vi "A170316-11-Main-large.vi"() -> ()   [LabVIEW 2020]
uses:
  System.Windows.Forms
  Database/Global1.vi
  Global_Variable/Global.vi
  <userlib>/_MGI/Menu Building/MenuItemStatusChange/MGI_MenuItemStatusChange.lvclass
panel:
  out "前序状态字":string
  out "前序状态":bool
  out "ECU自动":bool
  out "电机结果显示":string
  in  "质量报警":bool caption="布尔"
  in  "设备缺料":bool caption="布尔"
  in  "设备故障":bool caption="布尔"
  in  "设备离线":bool caption="布尔"
  in  "设备正常":bool caption="布尔"
  in  "菜单":refnum<k24>(container)
  out "检测结果":bool
  in  "批次信息":string[][](table)
  out "提示信息":string
  out "错误":bool
  out "时间字符串":string
  out "日期字符串":string
  out "电机自动":bool
  out "userStatus":string caption="用户状态"
  out "userName":string caption="用户名"
  out "生产数量":u32
  out "追溯码":string
  out "connectionMode":string caption="联机类型"
  out "产品型号":string
  in  "更换产品":refnum<vi>
  # "激光打标机"
  # "打标结果"
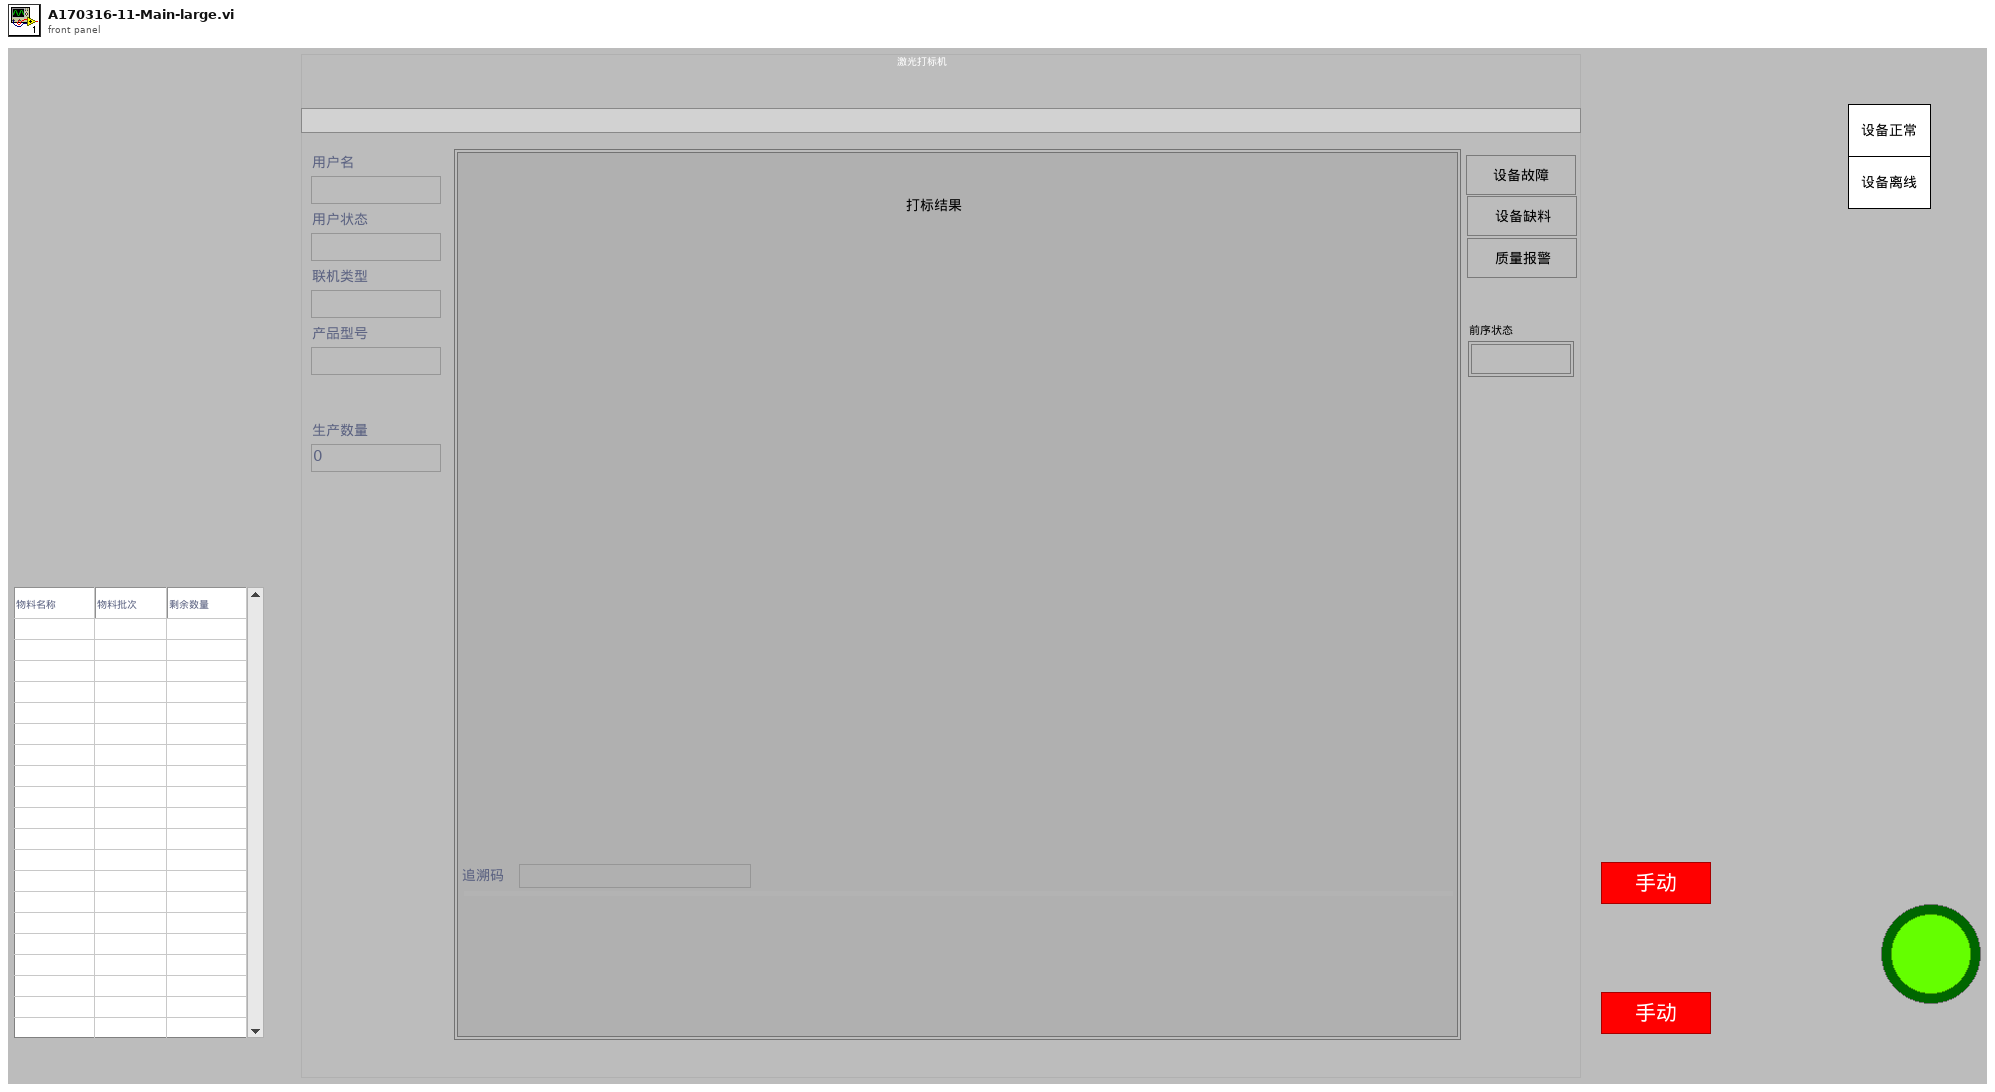
[diagram p1: front panel]
types:
  T1 = enum32{"Invalid", "Standard", "Closed", "Hidden", "Minimized", "Maximized"}
  T2 = enum32{"invalid app kind", "Development System", "Run Time System", "Student Edition", "Embedded LabVIEW", "Evaluation", "Custom"}
  T3 = cluster{"Core":cluster{"Current VI Reference":refnum<vi>, "Close Panel on Exit?":bool}, "Your Boolean data":bool, "Your string data":string}
  T4 = cluster{"Current VI Reference":refnum<vi>, "Close Panel on Exit?":bool}
  T5 = cluster{"用户编号":string, "用户名":string, "用户密码(密文)":string, "用户权限":string}
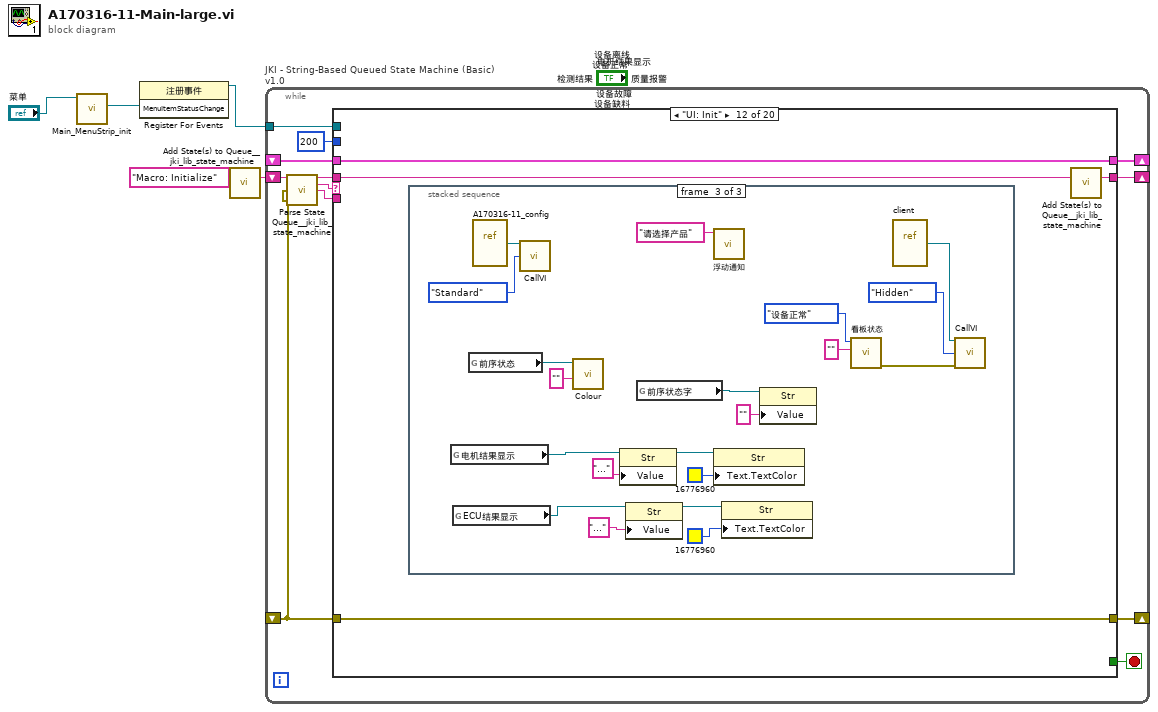
[diagram p0: block diagram]
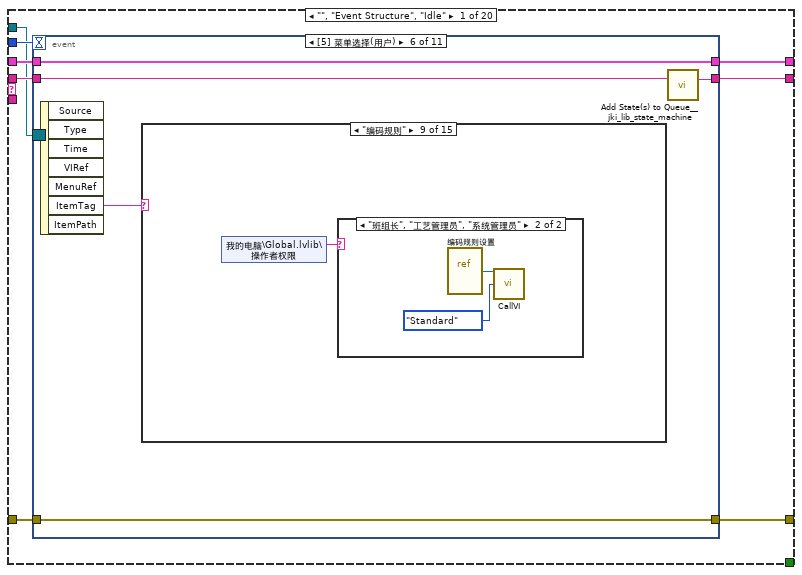
[diagram p2: hidden frame]
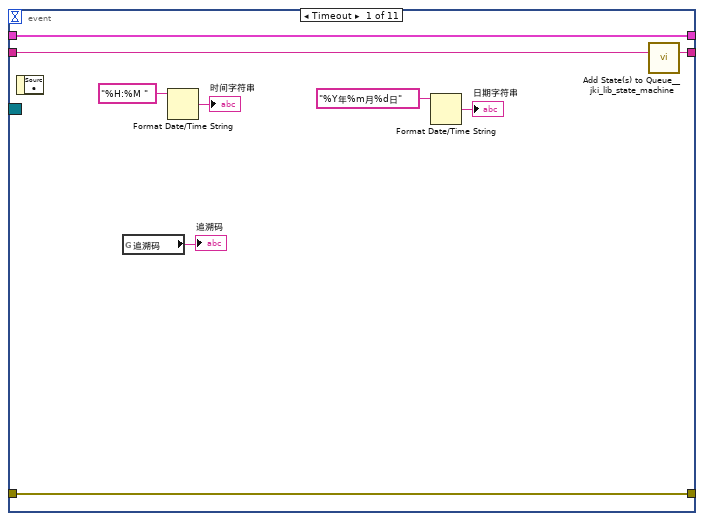
[diagram p3: hidden frame]
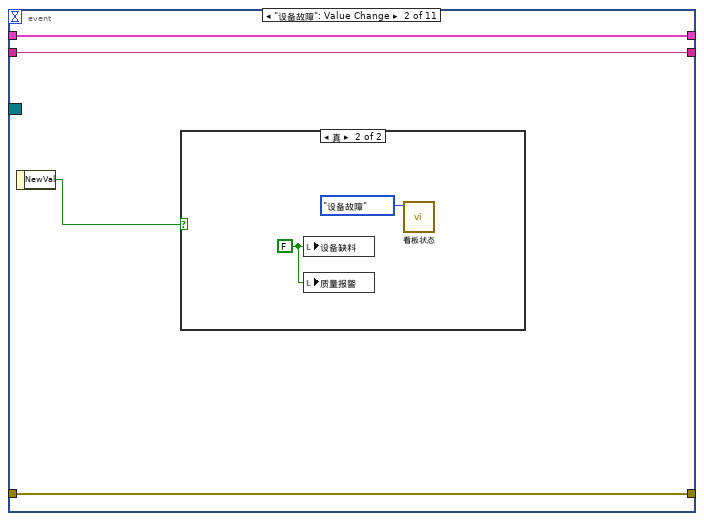
[diagram p4: hidden frame]
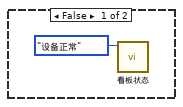
[diagram p5: hidden frame]
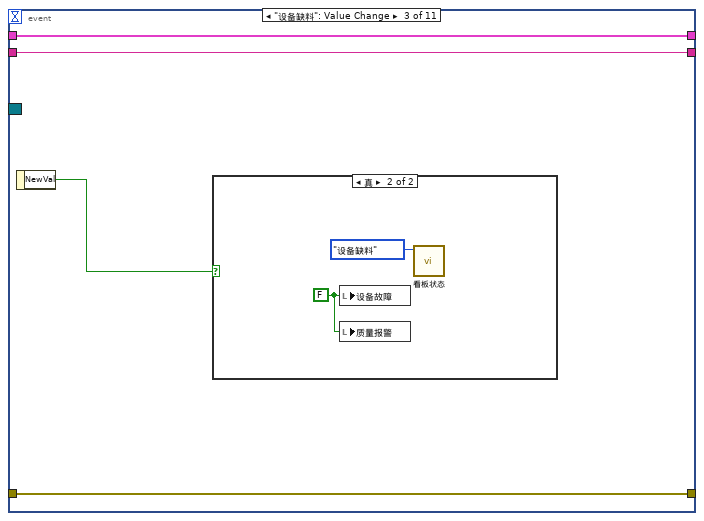
[diagram p6: hidden frame]
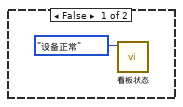
[diagram p7: hidden frame]
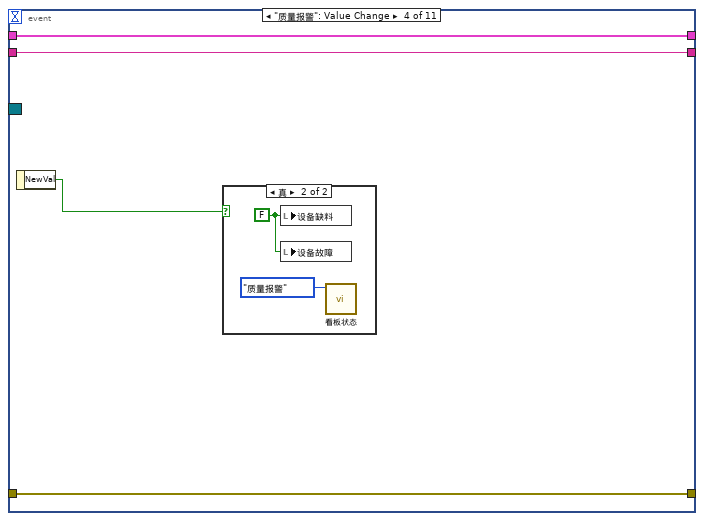
[diagram p8: hidden frame]
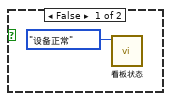
[diagram p9: hidden frame]
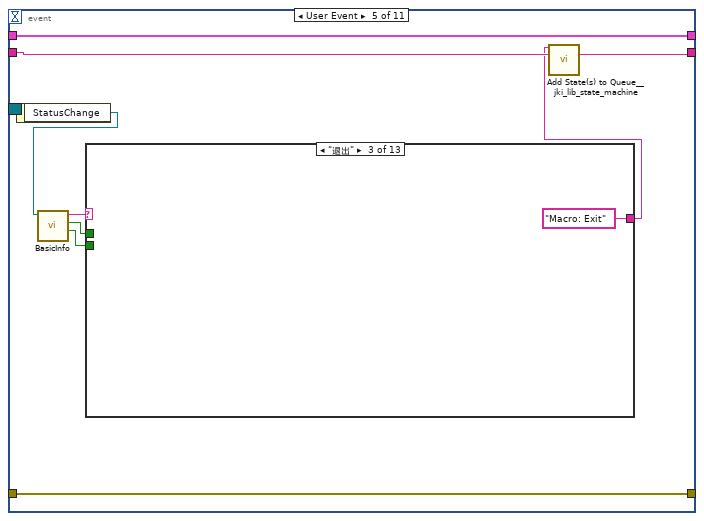
[diagram p10: hidden frame]
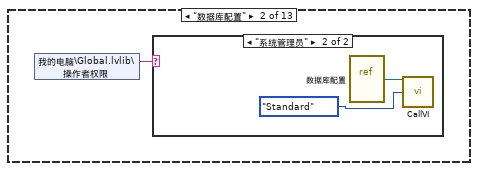
[diagram p12: hidden frame]
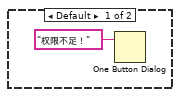
[diagram p13: hidden frame]
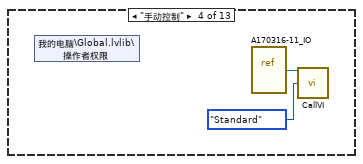
[diagram p14: hidden frame]
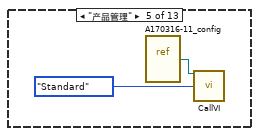
[diagram p15: hidden frame]
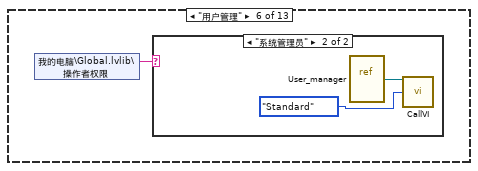
[diagram p16: hidden frame]
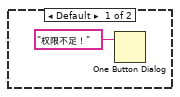
[diagram p17: hidden frame]
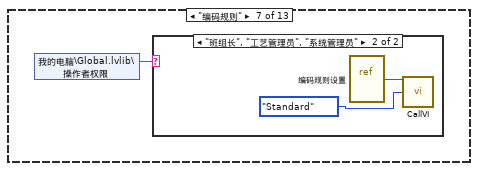
[diagram p18: hidden frame]
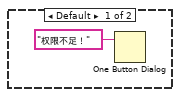
[diagram p19: hidden frame]
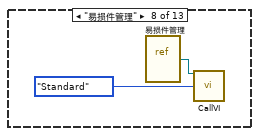
[diagram p20: hidden frame]
diagram:
  n1 = call "Main_MenuStrip_init.vi"("MenuStrip"="菜单") -> ("MenuItemStatusChange"=w2:refnum<user-event>)  [unwired: 9 in, 1 out]
  n2 = register-events(w2) -> (reference out=w1:refnum<event-registration>)  [unwired: 2 in, 1 out]
  n3 = call <vilib>:"Add State(s) to Queue__jki_lib_state_machine.vi"("State(s) in (\"\")"="Macro: Initialize") -> ("States Out"=w5:string)  [unwired: 14 in]
  n4 = while "JKI - String-Based Queued State Machine (Basic) v1.0" {
    shift-right: [w10] -> _
    shift-left: _ -> [w9]
    shift-right: [w13] -> _
    shift-left: _ -> [w7]
    shift-right: [w12] -> _
    shift-left: w5 -> [w14]
    tunnel: w1 -> [w6]
    stop <- w11 stop-if-true
    n5 = call <vilib>:"Parse State Queue__jki_lib_state_machine.vi"("State Queue"=w14, "Error In (no error)"=w7) -> ("Remaining States"=w16:string, "Current State"=w17:string, "Arguments"=w15:string)  [unwired: 11 in]
    n6 = case shown="\"UI: Init\"" w17 {
      selector: w17 -> [_ _ w202 _ _ _ _ _ _ _ _ _ _ _ _ _ _ _ _ _]
      tunnel: w16 -> [w25 w201 w206 w224 w230 w235 w239 w246 w252 w256 w268 w272 w319 w330 w356 w361 w374 w378 w382 w386]
      tunnel: w15 -> [_ _ _ _ _ _ _ _ _ _ _ _ w314 w324 _ _ _ _ _ _]
      tunnel: w9 -> [w23 w198 w204 w215 w227 w233 w236 _ w247 w253 w266 w270 w317 w326 w353 w358 w371 w375 w379 w383]
      tunnel: [w22 w199 w208 w221 errorcluster {"status"=FALSE, "code"=0, "source"=""} ("error out") w232 w237 w243 w248 w254 w263 w269 w315 w327 w354 w359 w372 w376 w380 w384] -> w13
      tunnel: w7 -> [w21 w199 w207 w221 w226 w232 w237 w243 w249 w254 w258 w269 w316 w328 w354 w359 w372 w376 w380 w384]
      tunnel: [w24 w200 w205 w223 w229 w234 w238 w245 w251 w255 w267 w271 w318 w329 w355 w360 w373 w377 w381 w385] -> w12
      tunnel: [_ _ _ _ _ TRUE _ _ _ _ _ _ _ _ _ _ _ _ _ _] -> w11
      tunnel: [w20 w198 w204 w222 w227 w233 w236 w244 w247 w253 w266 w270 w317 w326 w353 w358 w371 w375 w379 w383] -> w10
      tunnel: 200 ("Timeout") -> [w19 _ _ _ _ _ _ _ _ _ _ _ _ _ _ _ _ _ _ _]
      tunnel: w6 -> [w18 _ _ _ _ _ _ _ _ _ _ _ _ _ _ _ _ _ _ _]
      frame "", "Event Structure", "Idle" {
        n7 = event shown="[5] 菜单选择(用户)" {
          selector: w18 -> [_ _ _ _ _ _ _ _ _ _ _]
          dyn-events: _ -> [_ _ _ _ _ _ _ _ _ _ _]
          timeout: w19 -> [_ _ _ _ _ _ _ _ _ _ _]
          tunnel: w25 -> [w34 w37 w44 w51 w59 w105 w155 w161 w182 w191 w194]
          tunnel: [w33 w37 w44 w51 w58 w103 w156 w161 w182 w190 w195] -> w24
          tunnel: w23 -> [w31 w38 w45 w52 w60 w104 w157 w162 w183 w188 w197]
          tunnel: [w32 w36 w43 w50 w56 w106 w154 w160 w181 w189 w196] -> w22
          tunnel: w21 -> [w32 w36 w43 w50 w56 w106 w154 w160 w181 w189 w196]
          tunnel: [w31 w38 w45 w52 w60 w104 w157 w162 w183 w188 w197] -> w20
          event Timeout {
            n8 = event-data() -> ()  [unwired: 1 in, 1 out]
            n9 = global read "Global1.vi" "追溯码"() -> (→"追溯码":string)
            n10 = Format Date/Time String(time format string (%c)="%H:%M ") -> (date/time string=→"时间字符串":string)  [unwired: 2 in]
            n11 = Format Date/Time String(time format string (%c)="%Y年%m月%d日") -> (date/time string=→"日期字符串":string)  [unwired: 2 in]
            n12 = call <vilib>:"Add State(s) to Queue__jki_lib_state_machine.vi"("State(s) in (\"\")"=w34) -> ("States Out"=w33:string)  [unwired: 14 in]
          }
          event "设备故障": Value Change {
            n13 = event-data() -> ("NewVal"=w35:bool)  [unwired: 1 in]
            n14 = case shown="真" w35 {
              frame False {
                n15 = call "看板状态.vi"("设备状态"=enum16{"设备离线", "设备正常", "设备缺料", "设备故障", "质量报警"}."设备正常") -> ()  [unwired: 10 in, 1 out]
              }
              frame True {
                w40 = FALSE ("质量报警")
                n16 = local write "设备缺料"(w40) -> ()
                n17 = local write "质量报警"(w40) -> ()
                n18 = call "看板状态.vi"("设备状态"=enum16{"设备离线", "设备正常", "设备缺料", "设备故障", "质量报警"}."设备故障") -> ()  [unwired: 10 in, 1 out]
              }
            }
          }
          event "设备缺料": Value Change {
            n19 = event-data() -> ("NewVal"=w42:bool)  [unwired: 1 in]
            n20 = case shown="真" w42 {
              frame False {
                n21 = call "看板状态.vi"("设备状态"=enum16{"设备离线", "设备正常", "设备缺料", "设备故障", "质量报警"}."设备正常") -> ()  [unwired: 10 in, 1 out]
              }
              frame True {
                w47 = FALSE ("质量报警")
                n22 = local write "设备故障"(w47) -> ()
                n23 = local write "质量报警"(w47) -> ()
                n24 = call "看板状态.vi"("设备状态"=enum16{"设备离线", "设备正常", "设备缺料", "设备故障", "质量报警"}."设备缺料") -> ()  [unwired: 10 in, 1 out]
              }
            }
          }
          event "质量报警": Value Change {
            n25 = event-data() -> ("NewVal"=w49:bool)  [unwired: 1 in]
            n26 = case shown="真" w49 {
              frame False {
                n27 = call "看板状态.vi"("设备状态"=enum16{"设备离线", "设备正常", "设备缺料", "设备故障", "质量报警"}."设备正常") -> ()  [unwired: 10 in, 1 out]
              }
              frame True {
                w54 = FALSE ("质量报警")
                n28 = local write "设备缺料"(w54) -> ()
                n29 = local write "设备故障"(w54) -> ()
                n30 = call "看板状态.vi"("设备状态"=enum16{"设备离线", "设备正常", "设备缺料", "设备故障", "质量报警"}."质量报警") -> ()  [unwired: 10 in, 1 out]
              }
            }
          }
          event User Event {
            n31 = event-data() -> ("StatusChange"=w61:refnum<class "MGI_MenuItemStatusChange.lvclass">)  [unwired: 1 in]
            n32 = call <userlib>:"BasicInfo.vi"("MGI_MenuItemStatusChange in"=w61) -> ("Enabled?"=w64:bool, "Checked?"=w63:bool, "Tag"=w62:string)  [unwired: 7 in, 1 out]
            n33 = case shown="\"退出\"" w62 {
              tunnel: w63 -> [_ _ _ _ _ _ _ _ _ _ _ _ _]
              tunnel: w64 -> [_ _ _ _ _ _ _ _ _ _ _ _ _]
              tunnel: [_ _ "Macro: Exit" _ _ _ _ _ _ _ _ _ _] -> w57
              frame Default {
              }
              frame "数据库配置" {
                n34 = shared-variable "我的电脑\\Global.lvlib\\操作者权限"() -> (w65:string)  [unwired: 1 in, 1 out]
                n35 = case shown="\"系统管理员\"" w65 {
                  frame Default {
                    n36 = One Button Dialog(message="权限不足！" ("消息")) -> ()  [unwired: 1 in, 1 out]
                  }
                  frame "系统管理员" {
                    n37 = vi-ref "数据库配置.vi"() -> (w68:refnum<vi>)
                    n38 = call "CallVI.vi"("VI引用"=w68, "状态"=T1."Standard") -> ()  [unwired: 11 in, 3 out]
                  }
                }
              }
              frame "退出" {
              }
              frame "手动控制" {
                n39 = shared-variable "我的电脑\\Global.lvlib\\操作者权限"() -> ()  [unwired: 1 in, 2 out]
                n40 = vi-ref "A170316-11_IO.vi"() -> (w71:refnum<vi>)
                n41 = call "CallVI.vi"("VI引用"=w71, "状态"=T1."Standard") -> ()  [unwired: 11 in, 3 out]
              }
              frame "产品管理" {
                n42 = vi-ref "A170316-11_config.vi"() -> (w73:refnum<vi>)
                n43 = call "CallVI.vi"("VI引用"=w73, "状态"=T1."Standard") -> ()  [unwired: 11 in, 3 out]
              }
              frame "用户管理" {
                n44 = shared-variable "我的电脑\\Global.lvlib\\操作者权限"() -> (w74:string)  [unwired: 1 in, 1 out]
                n45 = case shown="\"系统管理员\"" w74 {
                  frame Default {
                    n46 = One Button Dialog(message="权限不足！" ("消息")) -> ()  [unwired: 1 in, 1 out]
                  }
                  frame "系统管理员" {
                    n47 = vi-ref "User_manager.vi"() -> (w77:refnum<vi>)
                    n48 = call "CallVI.vi"("VI引用"=w77, "状态"=T1."Standard") -> ()  [unwired: 11 in, 3 out]
                  }
                }
              }
              frame "编码规则" {
                n49 = shared-variable "我的电脑\\Global.lvlib\\操作者权限"() -> (w78:string)  [unwired: 1 in, 1 out]
                n50 = case shown="\"班组长\", \"工艺管理员\", \"系统管理员\"" w78 {
                  frame Default {
                    n51 = One Button Dialog(message="权限不足！" ("消息")) -> ()  [unwired: 1 in, 1 out]
                  }
                  frame "班组长", "工艺管理员", "系统管理员" {
                    n52 = vi-ref "编码规则设置.vi"() -> (w81:refnum<vi>)
                    n53 = call "CallVI.vi"("VI引用"=w81, "状态"=T1."Standard") -> ()  [unwired: 11 in, 3 out]
                  }
                }
              }
              frame "易损件管理" {
                n54 = vi-ref "易损件管理.vi"() -> (w83:refnum<vi>)
                n55 = call "CallVI.vi"("VI引用"=w83, "状态"=T1."Standard") -> ()  [unwired: 11 in, 3 out]
              }
              frame "物料批次管理" {
                n56 = vi-ref "批次管理.vi"() -> (w85:refnum<vi>)
                n57 = call "CallVI.vi"("VI引用"=w85, "状态"=T1."Standard") -> ()  [unwired: 11 in, 3 out]
              }
              frame "报表" {
                n58 = call "文件对话框2"("start path"=path "D:/report", "prompt"="打开报表", "pattern (all files)"="*.doc;*.docx", "pattern label"="Word 文档") -> ("selected path"=w86:path, "error out"=w87:errorcluster)  [unwired: 8 in, 2 out]
                n59 = case shown="无错误" w87 {
                  selector: w87 -> [w93 w95]
                  tunnel: w86 -> [w94 _]
                  frame No Error {
                    w92 = 1 items=["Normal", "Maximize", "Minimize"] ("cpubbs_WindowState")
                    n60 = call "Open_Word.vi"("File Path"=w94, "cpubbs_WindowState"=w92, "错误输入（无错误）"=w93) -> ()  [unwired: 12 in, 1 out]
                  }
                  frame Error {
                    n61 = call <vilib>:"Clear Errors.vi"("error in (no error)"=w95) -> ()  [unwired: 5 in, 2 out]
                  }
                }
              }
              frame "报警信息" {
                n62 = vi-ref "报警信息.vi"() -> (w97:refnum<vi>)
                n63 = call "CallVI.vi"("VI引用"=w97, "状态"=T1."Standard") -> ()  [unwired: 11 in, 3 out]
              }
              frame "关于" {
                n64 = vi-ref "About.vi"() -> (w99:refnum<vi>)
                n65 = call "CallVI.vi"("VI引用"=w99, "状态"=T1."Standard") -> ()  [unwired: 11 in, 3 out]
              }
              frame "操作演示" {
                n66 = call <vilib>:"Application Directory.vi"() -> ("Application Directory"=w102:path)
                n67 = Build Path(base path=w102, name or relative path="操作演示" ("名称或相对路径")) -> (appended path=w101:path)
                n68 = call "自动播放ppt.vi"("路径"=w101) -> ()  [unwired: 10 in, 1 out]
              }
            }
            n69 = call <vilib>:"Add State(s) to Queue__jki_lib_state_machine.vi"("State(s) in Front (\"\")"=w57, "State(s) in (\"\")"=w59) -> ("States Out"=w58:string)  [unwired: 13 in]
          }
          event Menu Selection (User) {
            n70 = event-data() -> ("ItemTag"=w107:string)  [unwired: 1 in, 6 out]
            n71 = case shown="\"编码规则\"" w107 {
              frame "假", Default {
              }
              frame "数据库配置" {
                n72 = shared-variable "我的电脑\\Global.lvlib\\操作者权限"() -> (w108:string)  [unwired: 1 in, 1 out]
                n73 = case shown="\"系统管理员\"" w108 {
                  frame Default {
                    n74 = One Button Dialog(message="权限不足！" ("消息")) -> ()  [unwired: 1 in, 1 out]
                  }
                  frame "系统管理员" {
                    n75 = vi-ref "数据库配置.vi"() -> (w111:refnum<vi>)
                    n76 = call "CallVI.vi"("VI引用"=w111, "状态"=T1."Standard") -> ()  [unwired: 11 in, 3 out]
                  }
                }
              }
              frame "退出" {
                n77 = Quit LabVIEW() -> ()  [unwired: 1 in]
              }
              frame "手动控制" {
                n78 = shared-variable "我的电脑\\Global.lvlib\\操作者权限"() -> (w112:string)  [unwired: 1 in, 1 out]
                n79 = case shown="\"班组长\", \"系统管理员\"" w112 {
                  frame Default {
                    n80 = One Button Dialog(message="权限不足！" ("消息")) -> ()  [unwired: 1 in, 1 out]
                  }
                  frame "班组长", "系统管理员" {
                    n81 = vi-ref "A170316-11_IO.vi"() -> (w115:refnum<vi>)
                    n82 = call "CallVI.vi"("VI引用"=w115, "状态"=T1."Standard") -> ()  [unwired: 11 in, 3 out]
                  }
                }
              }
              frame "半自动控制" {
                n83 = disable-structure shown="启用" {
                  frame Disabled {
                    n84 = shared-variable "我的电脑\\Global.lvlib\\操作者权限"() -> (w116:string)  [unwired: 1 in, 1 out]
                    n85 = case shown="\"班组长\", \"系统管理员\"" w116 {
                      frame Default {
                        n86 = One Button Dialog(message="权限不足！" ("消息")) -> ()  [unwired: 1 in, 1 out]
                      }
                      frame "班组长", "系统管理员" {
                        n87 = call "CallVI.vi"("VI引用"=refnum<vi> refnum, "状态"=T1."Maximized") -> ()  [unwired: 11 in, 3 out]
                      }
                    }
                  }
                  frame Enabled {
                    n88 = One Button Dialog(message="当前设备不具备半自动功能！" ("消息")) -> ()  [unwired: 1 in, 1 out]
                  }
                }
              }
              frame "产品管理" {
                n89 = vi-ref "A170316-11_config.vi"() -> (w122:refnum<vi>)
                n90 = call "CallVI.vi"("VI引用"=w122, "状态"=T1."Standard") -> ()  [unwired: 11 in, 3 out]
              }
              frame "系统配置" {
              }
              frame "用户管理" {
                n91 = shared-variable "我的电脑\\Global.lvlib\\操作者权限"() -> (w123:string)  [unwired: 1 in, 1 out]
                n92 = case shown="\"系统管理员\"" w123 {
                  frame Default {
                    n93 = One Button Dialog(message="权限不足！" ("消息")) -> ()  [unwired: 1 in, 1 out]
                  }
                  frame "系统管理员" {
                    n94 = vi-ref "User_manager.vi"() -> (w126:refnum<vi>)
                    n95 = call "CallVI.vi"("VI引用"=w126, "状态"=T1."Standard") -> ()  [unwired: 11 in, 3 out]
                  }
                }
              }
              frame "编码规则" {
                n96 = shared-variable "我的电脑\\Global.lvlib\\操作者权限"() -> (w127:string)  [unwired: 1 in, 1 out]
                n97 = case shown="\"班组长\", \"工艺管理员\", \"系统管理员\"" w127 {
                  frame Default {
                    n98 = One Button Dialog(message="权限不足！" ("消息")) -> ()  [unwired: 1 in, 1 out]
                  }
                  frame "班组长", "工艺管理员", "系统管理员" {
                    n99 = vi-ref "编码规则设置.vi"() -> (w130:refnum<vi>)
                    n100 = call "CallVI.vi"("VI引用"=w130, "状态"=T1."Standard") -> ()  [unwired: 11 in, 3 out]
                  }
                }
              }
              frame "易损件管理" {
                n101 = vi-ref "易损件管理.vi"() -> (w132:refnum<vi>)
                n102 = call "CallVI.vi"("VI引用"=w132, "状态"=T1."Standard") -> ()  [unwired: 11 in, 3 out]
              }
              frame "物料批次管理" {
                n103 = vi-ref "批次管理.vi"() -> (w134:refnum<vi>)
                n104 = call "CallVI.vi"("VI引用"=w134, "状态"=T1."Standard") -> ()  [unwired: 11 in, 3 out]
              }
              frame "打开报表" {
                n105 = call "文件对话框"("start path"=path "D:/report", "prompt"="打开报表", "pattern (all files)"="*.doc;*.docx", "pattern label"="Word 文档") -> ("selected path"=w135:path, "error out"=w136:errorcluster)  [unwired: 8 in, 2 out]
                n106 = case shown="无错误" w136 {
                  selector: w136 -> [w142 w144]
                  tunnel: w135 -> [w143 _]
                  frame No Error {
                    w141 = 1 items=["Normal", "Maximize", "Minimize"] ("cpubbs_WindowState")
                    n107 = call "Open_Word.vi"("File Path"=w143, "cpubbs_WindowState"=w141, "错误输入（无错误）"=w142) -> ()  [unwired: 12 in, 1 out]
                  }
                  frame Error {
                    n108 = call <vilib>:"Clear Errors.vi"("error in (no error)"=w144) -> ()  [unwired: 5 in, 2 out]
                  }
                }
              }
              frame "报警信息" {
                n109 = vi-ref "报警信息.vi"() -> (w146:refnum<vi>)
                n110 = call "CallVI.vi"("VI引用"=w146, "状态"=T1."Standard") -> ()  [unwired: 11 in, 3 out]
              }
              frame "关于" {
                n111 = vi-ref "About.vi"() -> (w148:refnum<vi>)
                n112 = call "CallVI.vi"("VI引用"=w148, "状态"=T1."Standard") -> ()  [unwired: 11 in, 3 out]
              }
              frame "操作演示" {
                n113 = call <vilib>:"Application Directory.vi"() -> ("Application Directory"=w151:path)
                n114 = Build Path(base path=w151, name or relative path="操作演示" ("名称或相对路径")) -> (appended path=w150:path)
                n115 = call "自动播放ppt.vi"("路径"=w150) -> ()  [unwired: 10 in, 1 out]
              }
            }
            n116 = call <vilib>:"Add State(s) to Queue__jki_lib_state_machine.vi"("State(s) in (\"\")"=w105) -> ("States Out"=w103:string)  [unwired: 14 in]
          }
          event "错误": Mouse Down {
            n117 = event-data() -> ()  [unwired: 1 in, 8 out]
            n118 = vi-ref "报警信息.vi"() -> (w153:refnum<vi>)
            n119 = call "CallVI.vi"("VI引用"=w153, "状态"=T1."Standard") -> ()  [unwired: 11 in, 3 out]
            n120 = call <vilib>:"Add State(s) to Queue__jki_lib_state_machine.vi"("State(s) in (\"\")"=w155) -> ("States Out"=w156:string)  [unwired: 14 in]
          }
          event "电机自动": Mouse Down {
            n121 = event-data() -> ("CtlRef"=w159:refnum<vi>)  [unwired: 1 in, 7 out]
            n122 = property class="Bool (严格)"(reference=w159) -> ("Value"=w158:bool)  [unwired: 1 in, 2 out]
            n123 = case shown="真" w158 {
              frame False {
                n124 = shared-variable "我的电脑\\JG.lvlib\\设备状态3"() -> (w163:i16)  [unwired: 1 in, 1 out]
                n125 = case shown="0, 默认" w163 {
                  frame 0, Default {
                    n126 = call "浮动通知.vi"("通知内容"="请复位！") -> ()  [unwired: 11 in]
                  }
                  frame 5 {
                    n127 = vi-ref "A170316-11_Auto.vi"() -> (w175:refnum<vi>)
                    n128 = invoke class="VI" method="Ctrl Val.Set"(reference=w175, "Control Name"="STEP3" ("控件名"), "Value"="初始化" ("控件名")) -> (reference out=w172:refnum<vi>, error out=w171:errorcluster)  [unwired: 2 in, 3 out]
                    n129 = invoke class="VI" method="Ctrl Val.Set"(reference=w172, error in=w171, "Control Name"="STEP2" ("控件名"), "Value"="初始化" ("控件名")) -> (reference out=w170:refnum<vi>, error out=w169:errorcluster)  [unwired: 1 in, 3 out]
                    n130 = invoke class="VI" method="Ctrl Val.Set"(reference=w170, error in=w169, "Control Name"="STEP1" ("控件名"), "Value"="初始化" ("控件名")) -> ()  [unwired: 1 in, 5 out]
                  }
                }
              }
              frame True {
                n131 = Two Button Dialog(message="自动程序运行中，\n是否切换为手动？" ("消息")) -> (T button?=w176:bool)  [unwired: 2 in]
                n132 = case shown="真" w176 {
                  frame False {
                  }
                  frame True {
                    n133 = vi-ref "A170316-11_Auto.vi"() -> (w180:refnum<vi>)
                    n134 = invoke class="VI" method="Ctrl Val.Set"(reference=w180, "Control Name"="STEP3" ("控件名"), "Value"="手动" ("控件名")) -> ()  [unwired: 2 in, 5 out]
                  }
                }
              }
            }
          }
          event "ECU自动": Mouse Down {
            n135 = event-data() -> ()  [unwired: 1 in, 8 out]
          }
          event Panel Close? {
            n136 = event-data() -> ()  [unwired: 1 in, 1 out]
            n137 = vi-ref "client.vi"() -> (w184:refnum<vi>)
            n138 = invoke class="VI" method="Abort VI"(reference=w184) -> ()  [unwired: 2 in, 3 out]
            n139 = global write "Global.vi" "程序关闭"(TRUE ("程序关闭")) -> ()
            n140 = event-data("Discard?"=TRUE) -> ()  [unwired: 1 in, 1 out]
            n141 = call <vilib>:"Add State(s) to Queue__jki_lib_state_machine.vi"("State(s) in Front (\"\")"="Macro: Exit", "State(s) in (\"\")"=w191) -> ("States Out"=w190:string)  [unwired: 13 in]
          }
          event "更换产品": Value Change {
            n142 = event-data() -> ("NewVal"=w193:refnum<vi>)  [unwired: 1 in, 5 out]
            n143 = control-ref of="子面板"() -> (w192:refnum<vi>)
            n144 = call "Call_SubPanal.vi"("VI引用句柄"=w193, "SubPnl引用句柄"=w192) -> ()  [unwired: 9 in, 1 out]
            n145 = call <vilib>:"Add State(s) to Queue__jki_lib_state_machine.vi"("State(s) in (\"\")"=w194) -> ("States Out"=w195:string)  [unwired: 14 in]
          }
        }
      }
      frame "---------- Core ----------" {
        n146 = call <vilib>:"Add State(s) to Queue__jki_lib_state_machine.vi"("State(s) in (\"\")"=w201) -> ("States Out"=w200:string)  [unwired: 14 in]
      }
      frame Default {
        w211 = 42 items=["No error", "Argument error", "Memory is full", "Out of zone", "End of file", "File already open", "Generic file I/O error", "File not found", "File permission error", "Disk is full", "Duplicate path", "Too many files open", "System feature not enabled", "Resource file not found", "Cannot add resource", "Resource not found", "Image not found", "Image memory error", "Pen does not exist", "Config type invalid", "Config token not found", "Config parse error", "Config memory error", "Bad external code format", "Bad external code offset", "External code not present", "Null window", "Destroy window error", "Null menu", "Print aborted", "Bad print record", "Print driver error", "Windows error during printing", "Memory error during printing", "Print dialog error", "Generic print error", "Invalid device refnum", "Device not found", "Device parameter error", "Device unit error", "Cannot open device", "Device call aborted", "Generic error", "Cancelled by user", "Object ID too low", "Object ID too high", "Object not in heap", "Unknown heap", "Unknown object (invalid DefProc)", "Unknown object (DefProc not in table)", "Message out of range", "Invalid (null) method", "Unknown message", "Manager call not supported", "Bad address", "Network operation in progress", "Network operation timed out", "Connection is busy", "Network attribute not supported", "Network error", "Address in use", "System out of memory", "Connection aborted", "Connection refused", "Not connected", "Already connected", "Connection closed", "Initialization error (interapplication manager)", "Bad occurrence", "Wait on unbound occurrence handler", "Occurrence queue overflow", "Datalog type conflict", "Unused", "Unrecognized type (interapplication manager)", "Memory corrupt", "Failed to make temporary DLL", "Old CIN version", "Drag socket not found", "Failed to load drop-object", "Failed to register OLE object", "Failed to release OLE object", "Format specifier type mismatch", "Unknown format specifier", "Too few format specifiers", "Too many format specifiers", "Scan failed", "Newer CIN version", "Error converting to variant", "Runtime menu error", "Password tampered", "Variant attribute not found", "Incompatible variant data type", "Event data is not available", "Event Store is not present", "Occurrence is not found", "Event Queue is not created", "Event info is not available", "Refnum passed is NULL", "Error retrieving Class GUID", "Error retrieving CoClass GUID", "Error retrieving TypeLib GUID.", "Bad built application magic bytes.", "Specific driver is different from the specific driver associated with the Logical Name.", "There is no session opened to the class driver.", "Max Error", "MAX - Error with config objects", "MAX - Error loading configuration", "MAX - Group not supported"]
        # "Current State"
        n147 = Format Into String(format string="Software Exception: Unhandled State \"%s\"." ("message"), error in=w207, w202) -> (resulting string=w210:string, error out=w209:errorcluster)  [unwired: 1 in]
        n148 = call <vilib>:"Error Cluster From Error Code.vi"("show call chain? (False)"=TRUE, "error in (no error)"=w209, "error message (\"\")"=w210, "error code (0)"=w211) -> ("error out"=w208:errorcluster)  [unwired: 5 in]
        n149 = call <vilib>:"Add State(s) to Queue__jki_lib_state_machine.vi"("State(s) in (\"\")"=w206) -> ("States Out"=w205:string)  [unwired: 14 in]
      }
      frame "Initialize Core Data" {
        # "originally closed?"
        # "exe?"
        n150 = property class="VI"() -> ("Front Panel.Open"=w220:bool)  [unwired: 2 in, 2 out]
        n151 = property class="App"() -> ("App.Kind"=w219:T2)  [unwired: 2 in, 2 out]
        n152 = control-ref of="Current VI Reference"() -> (w213:refnum<vi>)
        n153 = Not(x=w220) -> (.not. x?=w217:bool)
        n154 = Equal?(x=w219, y=T2."Run Time System" ("Application:Kind")) -> (x = y?=w216:bool)
        n155 = Or(x=w217, y=w216) -> (x .or. y?=w214:bool)
        n156 = Bundle By Name(cluster=w215, "Core.Current VI Reference"=w213, "Core.Close Panel on Exit?"=w214) -> (w222:T3)
        n157 = call <vilib>:"Add State(s) to Queue__jki_lib_state_machine.vi"("State(s) in (\"\")"=w224) -> ("States Out"=w223:string)  [unwired: 14 in]
      }
      frame "Error Handler" {
        n158 = call <vilib>:"General Error Handler.vi"("error in (no error)"=w226) -> ()  [unwired: 10 in, 5 out]
        n159 = call <vilib>:"Add State(s) to Queue__jki_lib_state_machine.vi"("State(s) in Front (\"\")"="/* Post Error States", "State(s) in (\"\")"=w230) -> ("States Out"=w229:string)  [unwired: 13 in]
      }
      frame "Exit" {
        n160 = call <vilib>:"Add State(s) to Queue__jki_lib_state_machine.vi"("State(s) in (\"\")"=w235) -> ("States Out"=w234:string)  [unwired: 14 in]
      }
      frame "---------- Data ----------" {
        n161 = call <vilib>:"Add State(s) to Queue__jki_lib_state_machine.vi"("State(s) in (\"\")"=w239) -> ("States Out"=w238:string)  [unwired: 14 in]
      }
      frame "Data: Initialize" {
        w240 = T4 {"Current VI Reference"=refnum, "Close Panel on Exit?"=FALSE}  # Core
        w242 = TRUE  # Your Boolean data
        w241 = ""  # Your string data
        n162 = Bundle("Core"=w240, "Your Boolean data"=w242, "Your string data"=w241) -> (w244:T3)  [unwired: 1 in]
        n163 = call <vilib>:"Add State(s) to Queue__jki_lib_state_machine.vi"("State(s) in (\"\")"=w246) -> ("States Out"=w245:string)  [unwired: 14 in]
      }
      frame "Data: Cleanup" {
        n164 = Unbundle By Name(w247) -> ("Core.Current VI Reference"=w250:refnum<vi>)
        n165 = Close Reference(reference=w250, error in (no error)=w249) -> (error out=w248:errorcluster)
        n166 = call <vilib>:"Add State(s) to Queue__jki_lib_state_machine.vi"("State(s) in (\"\")"=w252) -> ("States Out"=w251:string)  [unwired: 14 in]
      }
      frame "---------- UI ----------" {
        # "Do not put any code in this frame.\n(It is a separator no-op. You can make a copy of this frame to create a new UI frame)"
        n167 = call <vilib>:"Add State(s) to Queue__jki_lib_state_machine.vi"("State(s) in (\"\")"=w256) -> ("States Out"=w255:string)  [unwired: 14 in]
      }
      frame "UI: Initialize" {
        n168 = vi-ref "A170316-11_Auto.vi"() -> (w257:refnum<vi>)
        n169 = invoke on="子面板" class="SubPnl" method="Insert VI"(error in=w258, "VI Ref"=w257) -> (error out=w259:errorcluster)  [unwired: 2 in, 3 out]
        n170 = invoke class="VI" method="Run VI"(reference=w257, error in=w259, "Wait until done"=FALSE ("结束前等待"), "Auto Dispose Ref"=TRUE ("自动销毁引用")) -> (error out=w262:errorcluster)  [unwired: 1 in, 4 out]
        n171 = call "窗口自动调整.vi"("error in (no error)"=w262, "max？"=TRUE, "border spacing (2 px)"=0) -> ("error out"=w263:errorcluster)  [unwired: 3 in, 1 out]
        n172 = call <vilib>:"Add State(s) to Queue__jki_lib_state_machine.vi"("State(s) in (\"\")"=w268) -> ("States Out"=w267:string)  [unwired: 14 in]
      }
      frame "UI: Init" {
        n173 = stacked-sequence {
          frame #0 {
            n174 = shared-variable "我的电脑\\Global.lvlib\\联机模式"() -> (w279:i16)  [unwired: 1 in, 1 out]
            n175 = case shown="0, 默认" w279 {
              tunnel: ["联网" ("connectionMode") "单机" ("connectionMode")] -> w280
              frame 1 {
              }
              frame 0, Default {
              }
            }
            "connectionMode" <- w280
            n176 = global read "Global1.vi" "用户信息"() -> (w276:T5)
            n177 = Unbundle By Name(w276) -> ("用户权限"=w273:string, "用户名"=→"userName":string, "用户权限"=→"userStatus":string)
            n178 = shared-variable "我的电脑\\Global.lvlib\\操作者权限"(w273) -> ()  [unwired: 1 in, 1 out]
            "生产数量" <- u32 0 ("合格数量")
            "产品型号" <- "" ("productsName")
          }
          frame #1 {
            n179 = control-ref of="电机自动"() -> (w291:refnum<vi>)
            n180 = control-ref of="ECU自动"() -> (w285:refnum<vi>)
            n181 = control-ref of="更换产品"() -> (w289:refnum<vi>)
            n182 = global write "Global.vi" "电机程序自动"(w291) -> ()
            n183 = global write "Global.vi" "ECU自动"(w285) -> ()
            n184 = control-ref of="批次信息"() -> (w293:refnum<vi>)
            n185 = global write "Global.vi" "更换产品"(w289) -> ()
            n186 = global write "Global.vi" "批次"(w293) -> ()
            n187 = control-ref of="前序状态字"() -> (w284:refnum<vi>)
            n188 = control-ref of="前序状态"() -> (w283:refnum<vi>)
            n189 = control-ref of="错误"() -> (w292:refnum<vi>)
            n190 = global write "Global1.vi" "前序状态字"(w284) -> ()
            n191 = global write "Global.vi" "报警图标"(w292) -> ()
            n192 = global write "Global1.vi" "前序状态"(w283) -> ()
            n193 = control-ref of="提示信息"() -> (w290:refnum<vi>)
            n194 = control-ref of="生产数量"() -> (w288:refnum<vi>)
            n195 = control-ref of="电机结果显示"() -> (w286:refnum<vi>)
            n196 = control-ref of="检测结果"() -> (w287:refnum<vi>)
            n197 = global write "Global.vi" "安装支架生产数量"(w288) -> ()
            n198 = global write "Global.vi" "提示信息"(w290) -> ()
            n199 = global write "Global.vi" "检测结果"(w287) -> ()
            n200 = global write "Global.vi" "电机结果显示"(w286) -> ()
          }
          frame #2 {
            n201 = global read "Global.vi" "电机结果显示"() -> (w307:refnum<vi>)
            n202 = global read "Global.vi" "ECU结果显示"() -> (w300:refnum<vi>)
            n203 = global read "Global1.vi" "前序状态"() -> (w297:refnum<vi>)
            n204 = vi-ref "A170316-11_config.vi"() -> (w312:refnum<vi>)
            n205 = call "CallVI.vi"("VI引用"=w312, "状态"=T1."Standard") -> ()  [unwired: 11 in, 3 out]
            n206 = call "Colour.vi"("result"="", "colourRef"=w297) -> ()  [unwired: 9 in, 1 out]
            n207 = property class="Str"(reference=w307, "Value"="..." ("结果显示")) -> (reference out=w310:refnum<vi>)  [unwired: 1 in, 1 out]
            n208 = property class="Str"(reference=w300, "Value"="..." ("结果显示")) -> (reference out=w299:refnum<vi>)  [unwired: 1 in, 1 out]
            n209 = global read "Global1.vi" "前序状态字"() -> (w295:refnum<vi>)
            n210 = call "浮动通知.vi"("通知内容"="请选择产品") -> ()  [unwired: 11 in]
            n211 = property class="Str"(reference=w310, "Text.TextColor"=u32 16776960) -> ()  [unwired: 1 in, 2 out]
            n212 = property class="Str"(reference=w299, "Text.TextColor"=u32 16776960) -> ()  [unwired: 1 in, 2 out]
            n213 = property class="Str"(reference=w295, "Value"="" ("值")) -> ()  [unwired: 1 in, 2 out]
            n214 = call "看板状态.vi"("附加信息"="", "设备状态"=enum16{"设备离线", "设备正常", "设备缺料", "设备故障", "质量报警"}."设备正常") -> ("错误输出"=w302:errorcluster)  [unwired: 9 in]
            n215 = vi-ref "client.vi"() -> (w306:refnum<vi>)
            n216 = call "CallVI.vi"("VI引用"=w306, "状态"=T1."Hidden", "错误输入"=w302) -> ()  [unwired: 10 in, 3 out]
          }
        }
        n217 = call <vilib>:"Add State(s) to Queue__jki_lib_state_machine.vi"("State(s) in (\"\")"=w272) -> ("States Out"=w271:string)  [unwired: 14 in]
      }
      frame "UI: Cursor Set" {
        # "Argument"
        n218 = case shown="\"Idle\", 默认" w314 {
          tunnel: w316 -> [w321 w323]
          tunnel: [w320 w322] -> w315
          frame "Idle", Default {
            n219 = call <vilib>:"Unset Busy.vi"("error in (no error)"=w321) -> ("error out"=w320:errorcluster)  [unwired: 10 in]
          }
          frame "Busy" {
            n220 = call <vilib>:"Set Busy.vi"("error in (no error)"=w323) -> ("error out"=w322:errorcluster)  [unwired: 9 in, 1 out]
          }
        }
        n221 = call <vilib>:"Add State(s) to Queue__jki_lib_state_machine.vi"("State(s) in (\"\")"=w319) -> ("States Out"=w318:string)  [unwired: 14 in]
      }
      frame "UI: Front Panel State" {
        # "Argument"
        n222 = Unbundle By Name(w326) -> ("Core.Current VI Reference"=w325:refnum<vi>)
        n223 = case shown="\"Open\", 默认" w324 {
          tunnel: w328 -> [w334 w347]
          tunnel: [w336 w348] -> w327
          tunnel: w325 -> [w335 w345]
          frame "Open", Default {
            n224 = property class="VI"(reference=w335, error in=w334) -> (reference out=w332:refnum<vi>, error out=w333:errorcluster, "Front Panel.Open"=w331:bool)
            n225 = case shown="假" w331 {
              tunnel: [w339 w342] -> w336
              tunnel: w333 -> [w338 w342]
              tunnel: w332 -> [w337 _]
              frame False {
                n226 = invoke class="VI" method="FP.Open"(reference=w337, error in=w338, "Activate"=TRUE, "State"=T1."Standard") -> (error out=w339:errorcluster)  [unwired: 1 in, 4 out]
              }
              frame True {
              }
            }
          }
          frame "Close" {
            n227 = property class="VI"(reference=w345, error in=w347) -> (reference out=w344:refnum<vi>, error out=w346:errorcluster, "Front Panel.Open"=w343:bool)
            n228 = case shown="真" w343 {
              tunnel: [w349 w352] -> w348
              tunnel: w346 -> [w349 w351]
              tunnel: w344 -> [_ w350]
              frame False {
              }
              frame True {
                n229 = invoke class="VI" method="FP.Close"(reference=w350, error in=w351) -> (error out=w352:errorcluster)  [unwired: 1 in, 2 out]
              }
            }
          }
        }
        n230 = call <vilib>:"Add State(s) to Queue__jki_lib_state_machine.vi"("State(s) in (\"\")"=w330) -> ("States Out"=w329:string)  [unwired: 14 in]
      }
      frame "---------- Macro ----------" {
        n231 = call <vilib>:"Add State(s) to Queue__jki_lib_state_machine.vi"("State(s) in (\"\")"=w356) -> ("States Out"=w355:string)  [unwired: 14 in]
      }
      frame "Macro: Initialize" {
        w357 = "Data: Initialize\nInitialize Core Data\nUI: Initialize\nUI: Init\nUI: Front Panel State >> Open"  # Data: Initialize Initialize Core Data UI: Initialize UI: Init UI: Front Panel State >> Open
        n232 = call <vilib>:"Add State(s) to Queue__jki_lib_state_machine.vi"("State(s) in Front (\"\")"=w357, "State(s) in (\"\")"=w361) -> ("States Out"=w360:string)  [unwired: 13 in]
      }
      frame "Macro: Exit" {
        n233 = Unbundle By Name(w371) -> ("Core.Close Panel on Exit?"=w370:bool)
        n234 = vi-ref "client.vi"() -> (w364:refnum<vi>)
        n235 = invoke class="VI" method="FP.Close"(reference=w364) -> (reference out=w363:refnum<vi>, error out=w362:errorcluster)  [unwired: 2 in, 1 out]
        n236 = Close Reference(reference=w363, error in (no error)=w362) -> ()  [unwired: 1 out]
        n237 = Select(t="UI: Front Panel State >> Close", s=w370, f="") -> (s? t:f=w367:string)
        n238 = call <vilib>:"Add State(s) to Queue__jki_lib_state_machine.vi"("State(s) in (\"\")"=w367, "State(s) at Back (\"\")"="Data: Cleanup\nExit") -> ("States Out"=w365:string)  [unwired: 13 in]
        n239 = call <vilib>:"Add State(s) to Queue__jki_lib_state_machine.vi"("State(s) in Front (\"\")"=w365, "State(s) in (\"\")"=w374) -> ("States Out"=w373:string)  [unwired: 13 in]
      }
      frame "---------- New Category ----------" {
        n240 = call <vilib>:"Add State(s) to Queue__jki_lib_state_machine.vi"("State(s) in (\"\")"=w378) -> ("States Out"=w377:string)  [unwired: 14 in]
      }
      frame "New Category: 1" {
        n241 = call <vilib>:"Add State(s) to Queue__jki_lib_state_machine.vi"("State(s) in (\"\")"=w382) -> ("States Out"=w381:string)  [unwired: 14 in]
      }
      frame "New Category: 2" {
        n242 = call <vilib>:"Add State(s) to Queue__jki_lib_state_machine.vi"("State(s) in (\"\")"=w386) -> ("States Out"=w385:string)  [unwired: 14 in]
      }
    }
  }
